vi "IMAQdx_AbsImage_Flea3_v4.7.vi"() -> ()   [LabVIEW 2013] (continued)
rMOTpow3\tExpFinal(tEvap1,ODTpowX(DipPowX2),ODTpowX(DipPowX3),tau)\tfreq\tHeatingAmp\t0\tSine\tDetuning\tsingleFreqDet +20\tDoppCoolDet-DoppCoolSweep\tdopCoolT*1000\tDetuning\tsingleFreqStirDet + 20\tsingleFreqStirDet + SFramp + SFramp2\tloadT*1000\tBlueBN\tBlueLaserProbeBN\tSSteckBN\tShortSteckDDS\tPixisPos(TOF)\tCycle Wait for Move\t0\t0\t0\t0\t0\t0\t0\t0\t0\t0\t0\t0\t0\t0\t0\t0\t0\t0\t0\t0\t0\t0\t0\t0\r\npost evap hold\t\tRamp\t0\tholdT\t0\t0\t1\t1\t1\t1\t0\t0\t1\t1\t0\t0\t0\t1\t0\t0\t0\t1\t0\t0\t0\t0\t0\t0\t1m\t1\t1\t0\t0\t0\t1\t1\t0\tplus_zman\tminus_zman\tcompensation\trMOTcurrF\trMOTpow3\tcombAmplitude(combWidthF)\trMOTdelta(-(rMOTbroadDetuningF +combWidthF/2))\tODTpowHLat(DipPowHLat)\t0\t0\t0\t0\t1\t0\t1\t1\t0\tbMOTpow(0.5)\tProbePow\t0\tXshimrMOT\tYshimrMOT\tZshimVar\tODTpowZ(DipPowZ3)\t0\t0\tboxOn\t0\t0\t0\t0\t0\t0\t0\t0\t0\t0\t0\t0\t0\t0\t0\trMOTdelta(-(rMOTstirDetI +stirWidthF/2))\tODTpowBlue(BlueDipPow)\tExpFinal(tEvap1,ODTpowXY(DipPowCr2),ODTpowXY(DipPowCr3),tau)\tvarWaveP1\tProbePow2\tAmp688(depumpPow)\trMOTpow3\tExpFinal(tEvap1,ODTpowX(DipPowX2),ODTpowX(DipPowX3),tau)\tfreq\tHeatingAmp\t0\tSine\tDetuning\tsingleFreqDet +20\tDoppCoolDet-DoppCoolSweep\tdopCoolT*1000\tDetuning\tsingleFreqStirDet + 20\tsingleFreqStirDet + SFramp + SFramp2\tloadT*1000\tBlueBN\tBlueLaserProbeBN\tSSteckBN\tShortSteckDDS\tPixisPos(TOF)\tCycle Wait for Move\t0\t0\t0\t0\t0\t0\t0\t0\t0\t0\t0\t0\t0\t0\t0\t0\t0\t0\t0\t0\t0\t0\t0\t0\r\npost evap\t\tRamp\t0\tpulseLatT\t1\t1\t1\t1\t1\t1\t0\t0\t1\t1\t0\t0\t0\t1\t0\t0\t0\t1\t0\t0\t0\t0\t0\t0\t0\t1\t1\t0\t0\t0\t1\t1\t0\tplus_zman\tminus_zman\tcompensation\trMOTcurrF\trMOTpow3\tcombAmplitude(combWidthF)\trMOTdelta(-(rMOTbroadDetuningF +combWidthF/2))\tODTpowHLat(DipPowHLat2)\t0\t0\t0\t0\t1\t0\t1\t1\t0\tbMOTpow(0.5)\tProbePow\t0\tXshimrMOT\tYshimrMOT\tZshimVar\tODTpowZ(DipPowZ3)\t0\t0\t0\t0\t1\t1\t0\t0\t0\t0\t0\t0\t0\t0\t0\t0\t0\t0\trMOTdelta(-(rMOTstirDetI +stirWidthF/2))\tODTpowBlue(BlueDipPow)\tExpFinal(tEvap1,ODTpowXY(DipPowCr2),ODTpowXY(DipPowCr3),tau)\tvarWaveP1\tProbePow2\tAmp688(depumpPow)\trMOTpow3\tExpFinal(tEvap1,ODTpowX(DipPowX2),ODTpowX(DipPowX3),tau)\tfreq\tHeatingAmp\t0\tSine\tDetuning\tsingleFreqDet +20\tDoppCoolDet-DoppCoolSweep\tdopCoolT*1000\tDetuning\tsingleFreqStirDet + 20\tsingleFreqStirDet + SFramp + SFramp2\tloadT*1000\tBlueBN\tBlueLaserProbeBN\tSSteckBN\tShortSteckDDS\tPixisPos(TOF)\tCycle Wait for Move\t0\t0\t0\t0\t0\t0\t0\t0\t0\t0\t0\t0\t0\t0\t0\t0\t0\t0\t0\t0\t0\t0\t0\t0\r\npost evap hold\t\tRamp\t0\t2*rampLatT\t1\t1\t1\t1\t1\t1\t0\t0\t1\t1\t0\t0\t0\t1\t0\t0\t0\t1\t0\t0\t0\t0\t0\t0\t0\t1\t1\t0\t0\t0\t1\t1\t0\tplus_zman\tminus_zman\tcompensation\trMOTcurrF\trMOTpow3\tcombAmplitude(combWidthF)\trMOTdelta(-(rMOTbroadDetuningF +combWidthF/2))\tODTpowHLat(DipPowHLat)\t0\t0\t0\t0\t1\t0\t1\t1\t0\tbMOTpow(0.5)\tProbePow\t0\tXshimrMOT\tYshimrMOT\tZshimVar\tODTpowZ(DipPowZ3)\t0\t0\t0\t0\t1\t0\t0\t0\t0\t0\t0\t0\t0\t0\t0\t0\t0\t0\trMOTdelta(-(rMOTstirDetI +stirWidthF/2))\tODTpowBlue(BlueDipPow)\tExpFinal(tEvap1,ODTpowXY(DipPowCr2),ODTpowXY(DipPowCr3),tau)\tvarWaveP1\tProbePow2\tAmp688(depumpPow)\trMOTpow3\tExpFinal(tEvap1,ODTpowX(DipPowX2),ODTpowX(DipPowX3),tau)\tfreq\tHeatingAmp\t0\tSine\tDetuning\tsingleFreqDet +20\tDoppCoolDet-DoppCoolSweep\tdopCoolT*1000\tDetuning\tsingleFreqStirDet + 20\tsingleFreqStirDet + SFramp + SFramp2\tloadT*1000\tBlueBN\tBlueLaserProbeBN\tSSteckBN\tShortSteckDDS\tPixisPos(TOF)\tCycle Wait for Move\t0\t0\t0\t0\t0\t0\t0\t0\t0\t0\t0\t0\t0\t0\t0\t0\t0\t0\t0\t0\t0\t0\t0\t0\r\nlattice rampup\t\tRamp\t0\trampLatT\t1\t1\t1\t1\t1\t1\t0\t0\t1\t1\t0\t0\t0\t1\t0\t0\t0\t1\t0\t0\t0\t0\t0\t0\t10u\t1\t1\t0\t0\t0\t1\t1\t0\tplus_zman\tminus_zman\tcompensation\trMOTcurrF\trMOTpow3\tcombAmplitude(combWidthF)\trMOTdelta(-(rMOTbroadDetuningF +combWidthF/2))\tSinRamp(t,(ODTpowHLat(DipPowHLat)+ODTpowHLat(DipPowHLat2))/2,(ODTpowHLat(DipPowHLat)-ODTpowHLat(DipPowHLat2))/2,1/(2*rampLatT), pi/2)\t0\t0\t0\t0\t1\t0\t1\t1\t0\tbMOTpow(0.5)\tProbePow\t0\tXshimrMOT\tYshimrMOT\tZshimVar\tSinRamp(t,(ODTpowZ(DipPowZ3)+ODTpowZ(DipPowZLat))/2, (ODTpowZ(DipPowZ3)-ODTpowZ(DipPowZLat))/2, 1/(2*rampLatT), pi/2)\t0\t0\tboxOn\t0\t1\t1\t0\t0\t0\t0\t0\t0\t0\t0\t0\t0\t0\t0\trMOTdelta(-(rMOTstirDetI +stirWidthF/2))\tODTpowBlue(BlueDipPow)\tExpFinal(tEvap1,ODTpowXY(DipPowCr2),ODTpowXY(DipPowCr3),tau)\tLineRamp(f,varWaveP1,varWaveP2)\tProbePow2\tAmp688(depumpPow)\trMOTpow3\tExpFinal(tEvap1,ODTpowX(DipPowX2),ODTpowX(DipPowX3),tau)\tfreq\tHeatingAmp\t0\tSine\tDetuning\tsingleFreqDet +20\tDoppCoolDet-DoppCoolSweep\tdopCoolT*1000\tDetuning\tsingleFreqStirDet + 20\tsingleFreqStirDet + SFramp + SFramp2\tloadT*1000\tBlueBN\tBlueLaserProbeBN\tSSteckBN\tShortSteckDDS\tPixisPos(TOF)\tCycle Wait for Move\t0\t0\t0\t0\t0\t0\t0\t0\t0\t0\t0\t0\t0\t0\t0\t0\t0\t0\t0\t0\t0\t0\t0\t0\r\nODT rampdown\t\tRamp\t0\trampLatT\t1\t1\t1\t1\t1\t1\t0\t0\t1\t1\t0\t0\t0\t1\t0\t0\t0\t1\t0\t0\t0\t0\t0\t0\t1m\t1\t1\t0\t0\t0\t1\t1\t0\tplus_zman\tminus_zman\tcompensation\trMOTcurrF\trMOTpow3\tcombAmplitude(combWidthF)\trMOTdelta(-(rMOTbroadDetuningF +combWidthF/2))\tODTpowHLat(DipPowHLat2)\t0\t0\t0\t0\t1\t0\t1\t1\t0\tbMOTpow(0.5)\tProbePow\t0\tXshimrMOT\tYshimrMOT\tZshimVar\tODTpowZ(DipPowZLat)\t0\t0\tboxOn\t0\t1\t1\t0\t0\t0\t0\t0\t0\t0\t0\t0\t0\t0\t0\trMOTdelta(-(rMOTstirDetI +stirWidthF/2))\tODTpowBlue(BlueDipPow)\tSinRamp(t,(ExpFinal(tEvap1,ODTpowXY(DipPowCr2),ODTpowXY(DipPowCr3),tau)+ODTpowXY(0))/2,(ODTpowXY(0)-ExpFinal(tEvap1,ODTpowXY(DipPowCr2),ODTpowXY(DipPowCr3),tau))/2,1/(2*rampLatT),3*pi/2)\tvarWaveP2\tProbePow2\tAmp688(depumpPow)\trMOTpow3\tSinRamp(t,(ExpFinal(tEvap1,ODTpowX(DipPowX2),ODTpowX(DipPowX3),tau)+ODTpowX(0))/2,(ODTpowX(0)-ExpFinal(tEvap1,ODTpowX(DipPowX2),ODTpowX(DipPowX3),tau))/2,1/(2*rampLatT),3*pi/2)\tfreq\tHeatingAmp\t0\tSine\tDetuning\tsingleFreqDet +20\tDoppCoolDet-DoppCoolSweep\tdopCoolT*1000\tDetuning\tsingleFreqStirDet + 20\tsingleFreqStirDet + SFramp + SFramp2\tloadT*1000\tBlueBN\tBlueLaserProbeBN\tSSteckBN\tShortSteckDDS\tPixisPos(TOF)\tCycle Wait for Move\t0\t0\t0\t0\t0\t0\t0\t0\t0\t0\t0\t0\t0\t0\t0\t0\t0\t0\t0\t0\t0\t0\t0\t0\r\nlattice hold\t\tRamp\t0\t.1\t1\t1\t1\t1\t1\t1\t0\t0\t1\t1\t0\t0\t0\t1\t0\t0\t0\t1\t0\t0\t0\t0\t0\t0\t1m\t1\t1\t0\t0\t0\t1\t1\t0\tplus_zman\tminus_zman\tcompensation\trMOTcurrF\trMOTpow3\tcombAmplitude(combWidthF)\trMOTdelta(-(rMOTbroadDetuningF +combWidthF/2))\tODTpowHLat(DipPowHLat2)\t0\t0\t0\t0\t1\t0\t1\t1\t0\tbMOTpow(0.5)\tProbePow\t0\tXshimrMOT\tYshimrMOT\tZshimVar\tODTpowZ(DipPowZLat)\t0\t0\tboxOn\t0\t1\t1\t0\t0\t0\t0\t0\t0\t0\t0\t0\t0\t0\t0\trMOTdelta(-(rMOTstirDetI +stirWidthF/2))\tODTpowBlue(BlueDipPow)\tExpFinal(tEvap1,ODTpowXY(DipPowCr2),ODTpowXY(DipPowCr3),tau)\tvarWaveP2\tProbePow2\tAmp688(depumpPow)\trMOTpow3\tExpFinal(tEvap1,ODTpowX(DipPowX2),ODTpowX(DipPowX3),tau)\tfreq\tHeatingAmp\t0\tSine\tDetuning\tsingleFreqDet +20\tDoppCoolDet-DoppCoolSweep\tdopCoolT*1000\tDetuning\tsingleFreqStirDet + 20\tsingleFreqStirDet + SFramp + SFramp2\tloadT*1000\tBlueBN\tBlueLaserProbeBN\tSSteckBN\tShortSteckDDS\tPixisPos(TOF)\tCycle Wait for Move\t0\t0\t0\t0\t0\t0\t0\t0\t0\t0\t0\t0\t0\t0\t0\t0\t0\t0\t0\t0\t0\t0\t0\t0\r\nCross Beam Pulse\t\tRamp\t0\t.001\t1\t1\t1\t1\t1\t1\t0\t0\t1\t1\t0\t0\t0\t1\t0\t0\t0\t1\t0\t0\t0\t0\t0\t0\t1m\t1\t1\t0\t0\t0\t1\t1\t0\tplus_zman\tminus_zman\tcompensation\trMOTcurrF\trMOTpow3\tcombAmplitude(combWidthF)\trMOTdelta(-(rMOTbroadDetuningF +combWidthF/2))\tODTpowHLat(DipPowHLat2)\t0\t0\t0\t0\t1\t0\t1\t1\t0\tbMOTpow(0.5)\tProbePow\t0\tXshimrMOT\tYshimrMOT\tZshimVar\tODTpowZ(DipPowZLat)\t0\t0\tboxOn\t0\t1\t1\t0\t0\t0\t0\t0\t0\t0\t0\t0\t0\t0\t0\trMOTdelta(-(rMOTstirDetI +stirWidthF/2))\tODTpowBlue(BlueDipPow)\tODTpowXY(0.3)\tvarWaveP2\tProbePow2\tAmp688(depumpPow)\trMOTpow3\tExpFinal(tEvap1,ODTpowX(DipPowX2),ODTpowX(DipPowX3),tau)\tfreq\tHeatingAmp\t0\tSine\tDetuning\tsingleFreqDet +20\tDoppCoolDet-DoppCoolSweep\tdopCoolT*1000\tDetuning\tsingleFreqStirDet + 20\tsingleFreqStirDet + SFramp + SFramp2\tloadT*1000\tBlueBN\tBlueLaserProbeBN\tSSteckBN\tShortSteckDDS\tPixisPos(TOF)\tCycle Wait for Move\t0\t0\t0\t0\t0\t0\t0\t0\t0\t0\t0\t0\t0\t0\t0\t0\t0\t0\t0\t0\t0\t0\t0\t0\r\nbox ramp up\t\tRamp\t0\tboxLoadT\t1\t1\t1\t1\t1\t1\t0\t0\t1\t1\t0\t0\t0\t1\t0\t0\t0\t1\t0\t0\t0\t0\t0\t0\t1m\t1\t1\t0\t0\t0\t1\t1\t0\tplus_zman\tminus_zman\tcompensation\trMOTcurrF\trMOTpow3\tcombAmplitude(combWidthF)\trMOTdelta(-(rMOTbroadDetuningF +combWidthF/2))\tODTpowHLat(DipPowHLat2)\t0\t0\t0\t0\t1\t0\t1\t1\tpulseTTL(f,94)\tbMOTpow(0.5)\tProbePow\t0\tXshimrMOT\tYshimrMOT\tZshimVar\tODTpowZ(DipPowZ3)\t0\t0\tboxOn\t0\t1\t1\t0\t0\t0\t0\t0\t0\t0\t0\t0\t0\t0\t0\trMOTdelta(-(rMOTstirDetI +stirWidthF/2))\tSinRamp(t,(ODTpowBlue(BlueDipPow)+ODTpowBlue(0))/2,(ODTpowBlue(BlueDipPow)-ODTpowBlue(0))/2,1/(2*boxLoadT),3*pi/2)\tExpFinal(tEvap1,ODTpowXY(DipPowCr2),ODTpowXY(DipPowCr3),tau)\tvarWaveP1\tProbePow2\tAmp688(depumpPow)\trMOTpow3\tExpFinal(tEvap1,ODTpowX(DipPowX2),ODTpowX(DipPowX3),tau)\tfreq\tHeatingAmp\t0\tSine\tDetuning\tsingleFreqDet +20\tDoppCoolDet-DoppCoolSweep\tdopCoolT*1000\tDetuning\tsingleFreqStirDet + 20\tsingleFreqStirDet + SFramp + SFramp2\tloadT*1000\tBlueBN\tBlueLaserProbeBN\tSSteckBN\tShortSteckDDS\tPixisPos(TOF)\tCycle Wait for Move\t0\t0\t0\t0\t0\t0\t0\t0\t0\t0\t0\t0\t0\t0\t0\t0\t0\t0\t0\t0\t0\t0\t0\t0\r\npost evap hold\t\tRamp\t0\tholdT\t1\t1\t1\t1\t1\t1\t0\t0\t1\t1\t0\t0\t0\t1\t0\t0\t0\t1\t0\t0\t0\t0\t0\t0\t0\t1\t1\t0\t0\t0\t1\t1\t0\tplus_zman\tminus_zman\tcompensation\trMOTcurrF\trMOTpow3\tcombAmplitude(combWidthF)\trMOTdelta(-(rMOTbroadDetuningF +combWidthF/2))\tODTpowHLat(DipPowHLat2)\t0\t0\t0\t0\t1\t0\t1\t1\t0\tbMOTpow(0.5)\tProbePow\t0\tXshimrMOT\tYshimrMOT\tZshimVar\tODTpowZ(DipPowZLat)\t0\t0\tboxOn\t0\t1\t1\t0\t0\t0\t0\t0\t0\t0\t0\t0\t0\t0\t0\trMOTdelta(-(rMOTstirDetI +stirWidthF/2))\tODTpowBlue(BlueDipPow)\tExpFinal(tEvap1,ODTpowXY(DipPowCr2),ODTpowXY(DipPowCr3),tau)\tvarWaveP2\tProbePow2\tAmp688(depumpPow)\trMOTpow3\tExpFinal(tEvap1,ODTpowX(DipPowX2),ODTpowX(DipPowX3),tau)\tfreq\tHeatingAmp\t0\tSine\tDetuning\tsingleFreqDet +20\tDoppCoolDet-DoppCoolSweep\tdopCoolT*1000\tDetuning\tsingleFreqStirDet + 20\tsingleFreqStirDet + SFramp + SFramp2\tloadT*1000\tBlueBN\tBlueLaserProbeBN\tSSteckBN\tShortSteckDDS\tPixisPos(TOF)\tCycle Wait for Move\t0\t0\t0\t0\t0\t0\t0\t0\t0\t0\t0\t0\t0\t0\t0\t0\t0\t0\t0\t0\t0\t0\t0\t0\r\nlattice rampdown\t\tRamp\t0\trampLatOffT\t1\t1\t1\t1\t1\t1\t0\t0\t1\t1\t0\t0\t0\t1\t0\t0\t0\t1\t0\t0\t0\t0\t0\t0\t10u\t1\t1\t0\t0\t0\t1\t1\t0\tplus_zman\tminus_zman\tcompensation\trMOTcurrF\trMOTpow3\tcombAmplitude(combWidthF)\trMOTdelta(-(rMOTbroadDetuningF +combWidthF/2))\tSinRamp(t,(ODTpowHLat(DipPowHLat)+ODTpowHLat(DipPowHLat2))/2,(ODTpowHLat(DipPowHLat)-ODTpowHLat(DipPowHLat2))/2,1/(2*rampLatOffT), 3*pi/2)\t0\t0\t0\t0\t1\t0\t1\t1\t0\tbMOTpow(0.5)\tProbePow\t0\tXshimrMOT\tYshimrMOT\tZshimVar\tSinRamp(t,(ODTpowZ(DipPowZ3)+ODTpowZ(DipPowZLat))/2, (ODTpowZ(DipPowZ3)-ODTpowZ(DipPowZLat))/2, 1/(2*rampLatOffT), 3*pi/2)\t0\t0\t0\t0\t1\t1\t0\t0\t0\t0\t0\t0\t0\t0\t0\t0\t0\t0\trMOTdelta(-(rMOTstirDetI +stirWidthF/2))\tODTpowBlue(0)\tExpFinal(tEvap1,ODTpowXY(DipPowCr2),ODTpowXY(DipPowCr3),tau)\tLineRamp(f,varWaveP2,varWaveP1)\tProbePow2\tAmp688(depumpPow)\trMOTpow3\tExpFinal(tEvap1,ODTpowX(DipPowX2),ODTpowX(DipPowX3),tau)\tfreq\tHeatingAmp\t0\tSine\tDetuning\tsingleFreqDet +20\tDoppCoolDet-DoppCoolSweep\tdopCoolT*1000\tDetuning\tsingleFreqStirDet + 20\tsingleFreqStirDet + SFramp + SFramp2\tloadT*1000\tBlueBN\tBlueLaserProbeBN\tSSteckBN\tShortSteckDDS\tPixisPos(TOF)\tCycle Wait for Move\t0\t0\t0\t0\t0\t0\t0\t0\t0\t0\t0\t0\t0\t0\t0\t0\t0\t0\t0\t0\t0\t0\t0\t0\r\nEvaporation\t\tRamp\t0\ttEvap2\t1\t1\t1\t1\t1\t1\t0\t0\t1\t1\t0\t0\t0\t1\t0\t0\t0\t1\t0\t0\t0\t0\t0\t0\t50u\t1\t1\t0\t0\t0\t1\t1\t0\tplus_zman\tminus_zman\tcompensation\trMOTcurrF\trMOTpow3\tcombAmplitude(combWidthF)\trMOTdelta(-(rMOTbroadDetuningF +combWidthF/2))\tODTpowHLat(DipPowHLat)\t0\t0\t0\t0\t1\t0\t1\t1\t0\tbMOTpow(0.5)\tProbePow\t0\tXshimrMOT\tYshimrMOT\tZshimVar\tLineRamp(f,ODTpowZ(DipPowZ3),ODTpowZ(DipPowZ4))\t0\t0\t0\t0\t0\t1\t0\t0\t0\t0\t0\t0\t0\t0\t0\t0\t0\t0\trMOTdelta(-(rMOTstirDetI +stirWidthF/2))\tODTpowBlue(0)\tExpRamp2(t,0,ExpFinal(tEvap1,ODTpowXY(DipPowCr2),ODTpowXY(DipPowCr3),tau),ODTpowXY(DipPowCr4),tau2)\tvarWaveP1\tProbePow2\tAmp688(depumpPow)\trMOTpow3\tExpRamp2(t,0,ExpFinal(tEvap1,ODTpowX(DipPowX2),ODTpowX(DipPowX3),tau),ODTpowX(DipPowX4),tau2)\tfreq\tHeatingAmp\t0\tSine\tDetuning\tsingleFreqDet +20\tDoppCoolDet-DoppCoolSweep\tdopCoolT*1000\tDetuning\tsingleFreqStirDet + 20\tsingleFreqStirDet + SFramp + SFramp2\tloadT*1000\tBlueBN\tBlueLaserProbeBN\tSSteckBN\tShortSteckDDS\tPixisPos(TOF)\tCycle Wait for Move\t0\t0\t0\t0\t0\t0\t0\t0\t0\t0\t0\t0\t0\t0\t0\t0\t0\t0\t0\t0\t0\t0\t0\t0\r\npost evap hold\t\tRamp\t0\t.0075\t1\t1\t1\t1\t1\t1\t0\t0\t1\t1\t0\t0\t0\t1\t0\t0\t0\t1\t0\t0\t0\t0\t0\t0\t0\t1\t1\t0\t0\t0\t1\t1\t0\tplus_zman\tminus_zman\tcompensation\trMOTcurrF\trMOTpow3\tcombAmplitude(combWidthF)\trMOTdelta(-(rMOTbroadDetuningF +combWidthF/2))\tODTpowHLat(DipPowHLat)\t0\t0\t0\t0\t1\t0\t1\t1\t0\tbMOTpow(0.5)\tProbePow\t0\tXshimrMOT\tYshimrMOT\tZshimVar\tODTpowZ(DipPowZ4)\tVimaging\t0\t0\t0\t0\t1\t0\t0\t0\t0\t0\t0\t0\t0\t0\t0\t0\t0\trMOTdelta(-(rMOTstirDetI +stirWidthF/2))\tODTpowBlue(0)\tExpFinal(tEvap2,ODTpowXY(DipPowCr),ODTpowXY(DipPowCr2),tau)\tvarWaveP2\tProbePow2\tAmp688(depumpPow)\trMOTpow3\tExpFinal(tEvap1,ODTpowX(DipPowX),ODTpowX(DipPowX2),tau)\tfreq\tHeatingAmp\t0\tSine\tDetuning\tsingleFreqDet +20\tDoppCoolDet-DoppCoolSweep\tdopCoolT*1000\tDetuning\tsingleFreqStirDet + 20\tsingleFreqStirDet + SFramp + SFramp2\tloadT*1000\tBlueBN\tBlueLaserProbeBN\tSSteckBN\tShortSteckDDS\tPixisPos(TOF)\tCycle Wait for Move\t0\t0\t0\t0\t0\t0\t0\t0\t0\t0\t0\t0\t0\t0\t0\t0\t0\t0\t0\t0\t0\t0\t0\t0\r\nrMOT/Dip TOF\t\tRamp\t1\tTOFaux\t0\t0\t0\t0\t0\t0\t0\t0\t0\t1\t0\t0\t0\t0\t0\t0\t0\t1\t0\t0\t0\t0\t0\t0\t0\t1\t1\t0\t0\t0\t1\t1\t0\tplus_zman\tminus_zman\tcompensation\trMOTcurrF\trMOTpow5\tcombAmplitude(combWidthF)\trMOTdelta(-(rMOTbroadDetuningF +combWidthF/2))\tODTpowHLat(DipPowHLat2)\t0\tVimaging\t0\t0\t1\t0\t1\t1\t5\tbMOTpow(0.5)\tProbePow\t0\tXshimrMOT\tYshimrMOT\tZshimVar\tODTpowZ(DipPowZ4)\tVimaging\t0\t0\tHimaging\t0\t0\t0\t1\t0\t0\t0\t0\t0\t0\t0\t0\t0\t0\trMOTdelta(-(rMOTstirDetI +stirWidthF/2))\tODTpowBlue(0)\tODTpowXY(DipPowCrTOF)\tvarWaveP1\tProbePow2\tAmp688(depumpPow)\trMOTpow6\tODTpowX(DipPowXTOF)\tfreq\tHeatingAmp\t0\tSine\tDetuning\tsingleFreqDet +20\tDoppCoolDet-DoppCoolSweep\tdopCoolT*1000\tDetuning\tsingleFreqStirDet + 20\tsingleFreqStirDet + SFramp + SFramp2\tloadT*1000\tBlueBN\tBlueLaserProbeBN\tSSteckBN\tShortSteckDDS\tPixisPos(TOF)\tCycle Wait for Move\t0\t0\t0\t0\t0\t0\t0\t0\t0\t0\t0\t0\t0\t0\t0\t0\t0\t0\t0\t0\t0\t0\t0\t0\r\nBEC in situ\t\tRamp\t0\tTOFaux\t0\t0\t1\t1\t1\t1\t0\t0\t0\t1\t0\t0\t0\t0\t0\t0\t0\t1\t0\t0\t0\t0\t0\t0\t0\t1\t1\t0\t0\t0\t1\t1\t0\tplus_zman\tminus_zman\tcompensation\trMOTcurrF\trMOTpow5\tcombAmplitude(combWidthF)\trMOTdelta(-(rMOTbroadDetuningF +combWidthF/2))\tODTpowHLat(DipPowHLat)\t0\tVimaging\t0\t0\t1\t0\t1\t1\t0\tbMOTpow(0.5)\tProbePow\t0\tXshimrMOT\tYshimrMOT\tZshimVar\tODTpowZ(DipPowZ3)\tVimaging\t0\tboxOn\tHimaging\t0\t0\t0\t1\t0\t0\t0\t0\t0\t0\t0\t0\t0\t0\trMOTdelta(-(rMOTstirDetI +stirWidthF/2))\tODTpowBlue(.05)\tExpFinal(tEvap1,ODTpowXY(DipPowCr2),ODTpowXY(DipPowCr3),tau)\tvarWaveP1\tProbePow2\tAmp688(depumpPow)\trMOTpow6\tExpFinal(tEvap1,ODTpowX(DipPowX2),ODTpowX(DipPowX3),tau)\tfreq\tHeatingAmp\t0\tSine\tDetuning\tsingleFreqDet +20\tDoppCoolDet-DoppCoolSweep\tdopCoolT*1000\tDetuning\tsingleFreqStirDet + 20\tsingleFreqStirDet + SFramp + SFramp2\tloadT*1000\tBlueBN\tBlueLaserProbeBN\tSSteckBN\tShortSteckDDS\tPixisPos(TOF)\tCycle Wait for Move\t0\t0\t0\t0\t0\t0\t0\t0\t0\t0\t0\t0\t0\t0\t0\t0\t0\t0\t0\t0\t0\t0\t0\t0\r\nBEC in situ\t\tRamp\t0\tTOFaux\t0\t0\t0\t0\t0\t0\t0\t0\t0\t1\t0\t0\t0\t0\t0\t0\t0\t1\t0\t0\t0\t0\t0\t0\t0\t1\t1\t0\t0\t0\t1\t1\t0\tplus_zman\tminus_zman\tcompensation\trMOTcurrF\trMOTpow5\tcombAmplitude(combWidthF)\trMOTdelta(-(rMOTbroadDetuningF +combWidthF/2))\tODTpowHLat(DipPowHLat)\t0\tVimaging\t0\t0\t1\t0\t1\t1\t0\tbMOTpow(0.5)\tProbePow\t0\tXshimrMOT\tYshimrMOT\tZshimVar\tODTpowZ(DipPowZ3)\tVimaging\t0\tboxOn\tHimaging\t0\t0\t0\t1\t0\t0\t0\t0\t0\t0\t0\t0\t0\t0\trMOTdelta(-(rMOTstirDetI +stirWidthF/2))\tODTpowBlue(.05)\tExpFinal(tEvap1,ODTpowXY(DipPowCr2),ODTpowXY(DipPowCr3),tau)\tvarWaveP1\tProbePow2\tAmp688(depumpPow)\trMOTpow6\tExpFinal(tEvap1,ODTpowX(DipPowX2),ODTpowX(DipPowX3),tau)\tfreq\tHeatingAmp\t0\tSine\tDetuning\tsingleFreqDet +20\tDoppCoolDet-DoppCoolSweep\tdopCoolT*1000\tDetuning\tsingleFreqStirDet + 20\tsingleFreqStirDet + SFramp + SFramp2\tloadT*1000\tBlueBN\tBlueLaserProbeBN\tSSteckBN\tShortSteckDDS\tPixisPos(TOF)\tCycle Wait for Move\t0\t0\t0\t0\t0\t0\t0\t0\t0\t0\t0\t0\t0\t0\t0\t0\t0\t0\t0\t0\t0\t0\t0\t0\r\nLattice in situ\t\tRamp\t0\tTOFaux\t1\t1\t1\t1\t1\t1\t0\t0\t0\t1\t0\t0\t0\t0\t0\t0\t0\t1\t0\t0\t0\t0\t0\t0\t0\t1\t1\t0\t0\t0\t1\t1\t0\tplus_zman\tminus_zman\tcompensation\trMOTcurrF\trMOTpow5\tcombAmplitude(combWidthF)\trMOTdelta(-(rMOTbroadDetuningF +combWidthF/2))\tODTpowHLat(DipPowHLat2)\t0\tVimaging\t0\t0\t1\t0\t1\t1\t0\tbMOTpow(0.5)\tProbePow\t0\tXshimrMOT\tYshimrMOT\tZshimVar\tODTpowZ(DipPowZLat)\tVimaging\t0\tboxOn\tHimaging\t1\t1\t0\t0\t0\t0\t0\t0\t0\t0\t0\t0\t0\t0\trMOTdelta(-(rMOTstirDetI +stirWidthF/2))\tODTpowBlue(BlueDipPow)\tExpFinal(tEvap1,ODTpowXY(DipPowCr2),ODTpowXY(DipPowCr3),tau)\tvarWaveP2\tProbePow2\tAmp688(depumpPow)\trMOTpow6\tExpFinal(tEvap1,ODTpowX(DipPowX2),ODTpowX(DipPowX3),tau)\tfreq\tHeatingAmp\t0\tSine\tDetuning\tsingleFreqDet +20\tDoppCoolDet-DoppCoolSweep\tdopCoolT*1000\tDetuning\tsingleFreqStirDet + 20\tsingleFreqStirDet + SFramp + SFramp2\tloadT*1000\tBlueBN\tBlueLaserProbeBN\tSSteckBN\tShortSteckDDS\tPixisPos(TOF)\tCycle Wait for Move\t0\t0\t0\t0\t0\t0\t0\t0\t0\t0\t0\t0\t0\t0\t0\t0\t0\t0\t0\t0\t0\t0\t0\t0\r\nDipT in situ\t\tRamp\t0\tTOFaux\t1\t1\t1\t1\t1\t1\t0\t0\t0\t1\t0\t0\t0\t0\t0\t0\t0\t1\t0\t0\t0\t0\t0\t0\t0\t1\t1\t0\t0\t0\t1\t1\t0\tplus_zman\tminus_zman\tcompensation\trMOTcurrF\trMOTpow5\tcombAmplitude(combWidthF)\trMOTdelta(-(rMOTbroadDetuningF +combWidthF/2))\tODTpowHLat(DipPowHLat2)\t0\tVimaging\t0\t0\t1\t0\t1\t1\t0\tbMOTpow(0.5)\tProbePow\t0\tXshimrMOT\tYshimrMOT\tZshimVar\tODTpowZ(DipPowZFinal)\tVimaging\t0\tboxOn\tHimaging\t0\t1\t0\t0\t0\t0\t0\t0\t0\t0\t0\t0\t0\t0\trMOTdelta(-(rMOTstirDetI +stirWidthF/2))\tODTpowBlue(BlueDipPow)\tODTpowXY(DipPowCrFinal)\tvarWaveP1\tProbePow2\tAmp688(depumpPow)\trMOTpow6\tODTpowX(DipPowXFinal)\tfreq\tHeatingAmp\t0\tSine\tDetuning\tsingleFreqDet +20\tDoppCoolDet-DoppCoolSweep\tdopCoolT*1000\tDetuning\tsingleFreqStirDet + 20\tsingleFreqStirDet + SFramp + SFramp2\tloadT*1000\tBlueBN\tBlueLaserProbeBN\tSSteckBN\tShortSteckDDS\tPixisPos(TOF)\tCycle Wait for Move\t0\t0\t0\t0\t0\t0\t0\t0\t0\t0\t0\t0\t0\t0\t0\t0\t0\t0\t0\t0\t0\t0\t0\t0\r\nTOF\t\tRamp\t0\t.005\t1\t0\t0\t0\t0\t0\t0\t0\t0\t0\t0\t0\t0\t0\t0\t0\t0\t1\t0\t0\t0\t0\t0\t0\t0\t1\t1\t0\t0\t0\t1\t1\t0\tplus_zman\tminus_zman\tcompensation\trMOTcurrF\trMOTpow3\tcombAmplitude(combWidthF)\trMOTdelta(-(rMOTbroadDetuningF +combWidthF/2))\tODTpowHLat(DipPowHLat)\t0\tVimaging\t0\t0\t1\t0\t1\t1\t0\tbMOTpow(0.5)\tProbePow\t0\tXshimrMOT\tYshimrMOT\tZshimVar\tODTpowZ(DipPowZ)\tVimaging\t0\t0\tHimaging\t0\t0\t0\t0\t0\t0\t0\t0\t0\t0\t0\t0\t0\t0\trMOTdelta(-(rMOTstirDetI +stirWidthF/2))\tODTpowBlue(0)\tODTpowXY(DipPowCr)\tvarWaveP2\tProbePow2\tAmp688(depumpPow)\trMOTpow3\tODTpowX(DipPowX2)\tfreq\tHeatingAmp\t0\tSine\tDetuning\tsingleFreqDet +20\tDoppCoolDet-DoppCoolSweep\tdopCoolT*1000\tDetuning\tsingleFreqStirDet + 20\tsingleFreqStirDet + SFramp + SFramp2\tloadT*1000\tBlueBN\tBlueLaserProbeBN\tSSteckBN\tShortSteckDDS\tPixisPos(TOF)\tCycle Wait for Move\t0\t0\t0\t0\t0\t0\t0\t0\t0\t0\t0\t0\t0\t0\t0\t0\t0\t0\t0\t0\t0\t0\t0\t0\r\nTOF\t\tRamp\t1-rMOTon\t.001\t0\t0\t0\t0\t0\t0\t0\t0\t0\t0\t0\t0\t0\t0\t0\t0\t0\t1\t0\t0\t0\t0\t0\t0\t0\t1\t1\t0\t0\t0\t1\t1\t0\tplus_zman\tminus_zman\tcompensation\trMOTcurrF\trMOTpow3\tcombAmplitude(combWidthF)\trMOTdelta(-(rMOTbroadDetuningF +combWidthF/2))\t